vi "Dresden R2R Sputter 03.02.2018 IY24.vi"() -> ()   [LabVIEW 2009] (continued)
                                }
                                }
                                n17668 = local read "Semi"() -> (w26061:bool)
                                n17669 = Or(x=w26062, y=w26061) -> (x .or. y?=w26060:bool)
                                }
                                }
                                frame #1 {
                                }
                                }
                                }
                                frame #1 {
                                n17670 = local read "Semi"() -> (w26073:bool)
                                n17671 = case shown="False" w26073 {
                                frame #0 {
                                n17672 = local write "Ch2_PA7"(TRUE ("PA3")) -> ()
                                n17673 = Wait Until Next ms Multiple(millisecond multiple=u32 1000) -> ()  [unwired: 1 out]
                                }
                                frame #1 {
                                }
                                }
                                }
                                }
                              }
                              frame #1 {
                              }
                            }
                          }
                          frame #2 {
                            # "CLOSE BG-BV"
                            n17674 = local read "Semi"() -> (w26076:bool)
                            n17675 = case shown="False" w26076 {
                              frame #0 {
                                n17676 = stacked-sequence {
                                frame #0 {
                                n17677 = local read "Semi"() -> (w26077:bool)
                                n17678 = case shown="False" w26077 {
                                frame #0 {
                                n17679 = while {
                                i -> [w26084]
                                stop <- w26078 stop-if-true
                                n17680 = Greater?(x=w26084, y=50) -> (0:w26082:bool)
                                n17681 = case shown="True" w26082 {
                                frame #0 {
                                }
                                frame #1 {
                                n17682 = local write "Semi"(TRUE ("Semi")) -> ()
                                n17683 = local write "Error Message"("Start up process  cancelled\nbecause  BG-BV not closed.\nPlease check  BG-BV2 connections." ("Error Message")) -> ()
                                }
                                }
                                n17684 = local read "Ch2_Bg_bv_di"() -> (w26081:bool)
                                n17685 = case shown="True" w26081 {
                                tunnel: [TRUE FALSE] -> w26080
                                frame #0 {
                                }
                                frame #1 {
                                n17686 = Wait Until Next ms Multiple(millisecond multiple=u32 200) -> ()  [unwired: 1 out]
                                n17687 = local write "Ch2_Bg_bv_do"(FALSE ("Ch1_Tp_bv_do")) -> ()
                                }
                                }
                                n17688 = local read "Semi"() -> (w26079:bool)
                                n17689 = Or(x=w26080, y=w26079) -> (x .or. y?=w26078:bool)
                                }
                                }
                                frame #1 {
                                }
                                }
                                }
                                frame #1 {
                                n17690 = local read "Semi"() -> (w26091:bool)
                                n17691 = case shown="False" w26091 {
                                frame #0 {
                                n17692 = local write "Ch2_PA8"(TRUE ("PA3")) -> ()
                                n17693 = Wait Until Next ms Multiple(millisecond multiple=u32 1000) -> ()  [unwired: 1 out]
                                }
                                frame #1 {
                                }
                                }
                                }
                                }
                              }
                              frame #1 {
                              }
                            }
                          }
                          frame #3 {
                            # "CLOSE TP-BV"
                            n17694 = local read "Semi"() -> (w26094:bool)
                            n17695 = case shown="False" w26094 {
                              frame #0 {
                                n17696 = stacked-sequence {
                                frame #0 {
                                n17697 = local read "Semi"() -> (w26095:bool)
                                n17698 = case shown="False" w26095 {
                                frame #0 {
                                n17699 = while {
                                i -> [w26102]
                                stop <- w26096 stop-if-true
                                n17700 = Greater?(x=w26102, y=50) -> (0:w26100:bool)
                                n17701 = case shown="True" w26100 {
                                frame #0 {
                                }
                                frame #1 {
                                n17702 = local write "Semi"(TRUE ("Semi")) -> ()
                                n17703 = local write "Error Message"("Start up process  cancelled\nbecause  TP-BV not closed.\nPlease check  TP2-BV connections." ("Error Message")) -> ()
                                }
                                }
                                n17704 = local read "Ch2_Tp_bv_di"() -> (w26099:bool)
                                n17705 = case shown="True" w26099 {
                                tunnel: [TRUE FALSE] -> w26098
                                frame #0 {
                                }
                                frame #1 {
                                n17706 = Wait Until Next ms Multiple(millisecond multiple=u32 200) -> ()  [unwired: 1 out]
                                n17707 = local write "Ch2_Tp_bv_do"(FALSE ("Ch1_Tp_bv_do")) -> ()
                                }
                                }
                                n17708 = local read "Semi"() -> (w26097:bool)
                                n17709 = Or(x=w26098, y=w26097) -> (x .or. y?=w26096:bool)
                                }
                                }
                                frame #1 {
                                }
                                }
                                }
                                frame #1 {
                                n17710 = local read "Semi"() -> (w26109:bool)
                                n17711 = case shown="False" w26109 {
                                frame #0 {
                                n17712 = local write "Ch2_PA9"(TRUE ("PA5")) -> ()
                                n17713 = Wait Until Next ms Multiple(millisecond multiple=u32 1000) -> ()  [unwired: 1 out]
                                }
                                frame #1 {
                                }
                                }
                                }
                                }
                              }
                              frame #1 {
                              }
                            }
                          }
                          frame #4 {
                            # "False PL1-ATM"
                            n17714 = local read "Semi"() -> (w26112:bool)
                            n17715 = case shown="False" w26112 {
                              frame #0 {
                                n17716 = stacked-sequence {
                                frame #0 {
                                n17717 = local read "Semi"() -> (w26113:bool)
                                n17718 = case shown="False" w26113 {
                                frame #0 {
                                n17719 = local write "Ch2_Pl_atm_do"(FALSE ("Ch1_Pl_atm_do")) -> ()
                                }
                                frame #1 {
                                }
                                }
                                }
                                frame #1 {
                                n17720 = local read "Semi"() -> (w26115:bool)
                                n17721 = case shown="False" w26115 {
                                frame #0 {
                                n17722 = local write "Ch2_PA10"(TRUE ("PA3")) -> ()
                                n17723 = Wait Until Next ms Multiple(millisecond multiple=u32 1000) -> ()  [unwired: 1 out]
                                }
                                frame #1 {
                                }
                                }
                                }
                                }
                              }
                              frame #1 {
                              }
                            }
                          }
                          frame #5 {
                            # "STOP MP"
                            n17724 = local read "Semi"() -> (w26118:bool)
                            n17725 = case shown="False" w26118 {
                              frame #0 {
                                n17726 = stacked-sequence {
                                frame #0 {
                                n17727 = local read "Semi"() -> (w26119:bool)
                                n17728 = case shown="False" w26119 {
                                frame #0 {
                                n17729 = while {
                                i -> [w26126]
                                stop <- w26120 stop-if-true
                                n17730 = Greater?(x=w26126, y=50) -> (0:w26124:bool)
                                n17731 = case shown="True" w26124 {
                                frame #0 {
                                }
                                frame #1 {
                                n17732 = local write "Semi"(TRUE ("Semi")) -> ()
                                n17733 = local write "Error Message"("Start up process  cancelled\nbecause MP2 not stopped.\nPlease check MP2 connections." ("Error Message")) -> ()
                                }
                                }
                                n17734 = local read "Ch2_Mp_di"() -> (w26123:bool)
                                n17735 = case shown="True" w26123 {
                                tunnel: [TRUE FALSE] -> w26122
                                frame #0 {
                                }
                                frame #1 {
                                n17736 = Wait Until Next ms Multiple(millisecond multiple=u32 200) -> ()  [unwired: 1 out]
                                n17737 = local write "Ch2_Mp_do"(FALSE ("Ch1_Tp_bv_do")) -> ()
                                }
                                }
                                n17738 = local read "Semi"() -> (w26121:bool)
                                n17739 = Or(x=w26122, y=w26121) -> (x .or. y?=w26120:bool)
                                }
                                }
                                frame #1 {
                                }
                                }
                                }
                                frame #1 {
                                n17740 = local read "Semi"() -> (w26133:bool)
                                n17741 = case shown="False" w26133 {
                                frame #0 {
                                n17742 = local write "Ch2_PA11"(TRUE ("PA3")) -> ()
                                n17743 = Wait Until Next ms Multiple(millisecond multiple=u32 1000) -> ()  [unwired: 1 out]
                                }
                                frame #1 {
                                }
                                }
                                }
                                }
                              }
                              frame #1 {
                              }
                            }
                          }
                          frame #6 {
                            # "OPEN PL-VBV"
                            n17744 = local read "Semi"() -> (w26136:bool)
                            n17745 = case shown="False" w26136 {
                              frame #0 {
                                n17746 = stacked-sequence {
                                frame #0 {
                                n17747 = local read "Semi"() -> (w26137:bool)
                                n17748 = case shown="False" w26137 {
                                frame #0 {
                                n17749 = while {
                                i -> [w26144]
                                stop <- w26139 stop-if-true
                                n17750 = Greater?(x=w26144, y=50) -> (0:w26142:bool)
                                n17751 = case shown="True" w26142 {
                                frame #0 {
                                }
                                frame #1 {
                                n17752 = local write "Semi"(TRUE ("Semi")) -> ()
                                n17753 = local write "Error Message"("Start up process  cancelled\nbecause  PL-VBV not opened.\nPlease check PL-VBV2 connections." ("Error Message")) -> ()
                                }
                                }
                                n17754 = local read "Ch2_Pl_atm_di"() -> (w26138:bool)
                                n17755 = case shown="False" w26138 {
                                tunnel: [w26146 TRUE] -> w26141
                                frame #0 {
                                n17756 = local read "Ch2_Pl_vbv_di"() -> (w26145:bool)
                                n17757 = case shown="False" w26145 {
                                tunnel: [FALSE TRUE] -> w26146
                                frame #0 {
                                n17758 = Wait Until Next ms Multiple(millisecond multiple=u32 200) -> ()  [unwired: 1 out]
                                n17759 = local write "Ch2_Pl_vbv_do"(TRUE ("Ch1_Tp_bv_do")) -> ()
                                }
                                frame #1 {
                                }
                                }
                                }
                                frame #1 {
                                }
                                }
                                n17760 = local read "Semi"() -> (w26140:bool)
                                n17761 = Or(x=w26141, y=w26140) -> (x .or. y?=w26139:bool)
                                }
                                }
                                frame #1 {
                                }
                                }
                                }
                                frame #1 {
                                n17762 = local read "Semi"() -> (w26154:bool)
                                n17763 = case shown="False" w26154 {
                                frame #0 {
                                n17764 = local write "Ch2_PA12"(TRUE ("PA3")) -> ()
                                n17765 = Wait Until Next ms Multiple(millisecond multiple=u32 1000) -> ()  [unwired: 1 out]
                                }
                                frame #1 {
                                }
                                }
                                }
                                }
                              }
                              frame #1 {
                              }
                            }
                          }
                          frame #7 {
                            # "CHECK PL-PRESSURE"
                            n17766 = local read "Semi"() -> (w26157:bool)
                            n17767 = case shown="False" w26157 {
                              frame #0 {
                                n17768 = stacked-sequence {
                                frame #0 {
                                n17769 = local read "Semi"() -> (w26158:bool)
                                n17770 = case shown="False" w26158 {
                                frame #0 {
                                n17771 = while {
                                i -> [w26165]
                                stop <- w26160 stop-if-true
                                n17772 = Greater?(x=w26165, y=50) -> (0:w26163:bool)
                                n17773 = case shown="True" w26163 {
                                frame #0 {
                                }
                                frame #1 {
                                n17774 = local write "Semi"(TRUE ("Semi")) -> ()
                                n17775 = local write "Error Message"("Start up process  cancelled\nbecause  PL-ATM not opened.\nPlease check PL-ATM2 connections." ("Error Message")) -> ()
                                }
                                }
                                n17776 = local read "Ch2_Pl_atm_di"() -> (w26159:bool)
                                n17777 = case shown="True" w26159 {
                                tunnel: [FALSE TRUE] -> w26162
                                frame #0 {
                                }
                                frame #1 {
                                n17778 = Wait Until Next ms Multiple(millisecond multiple=u32 500) -> ()  [unwired: 1 out]
                                }
                                }
                                n17779 = local read "Semi"() -> (w26161:bool)
                                n17780 = Or(x=w26162, y=w26161) -> (x .or. y?=w26160:bool)
                                }
                                }
                                frame #1 {
                                }
                                }
                                }
                                frame #1 {
                                n17781 = local read "Semi"() -> (w26171:bool)
                                n17782 = case shown="False" w26171 {
                                frame #0 {
                                n17783 = local write "Ch2_PA13"(TRUE ("PA3")) -> ()
                                n17784 = Wait Until Next ms Multiple(millisecond multiple=u32 1000) -> ()  [unwired: 1 out]
                                }
                                frame #1 {
                                }
                                }
                                }
                                }
                              }
                              frame #1 {
                              }
                            }
                          }
                          frame #8 {
                            # "False CH-ATM"
                            n17785 = local read "Semi"() -> (w26174:bool)
                            n17786 = case shown="False" w26174 {
                              frame #0 {
                                n17787 = stacked-sequence {
                                frame #0 {
                                n17788 = local read "Semi"() -> (w26175:bool)
                                n17789 = case shown="False" w26175 {
                                frame #0 {
                                n17790 = local write "Ch2_Ch_atm_do"(FALSE ("Ch1_Pl_atm_do")) -> ()
                                }
                                frame #1 {
                                }
                                }
                                }
                                frame #1 {
                                n17791 = local read "Semi"() -> (w26177:bool)
                                n17792 = case shown="False" w26177 {
                                frame #0 {
                                n17793 = local write "Ch2_PA14"(TRUE ("PA3")) -> ()
                                n17794 = Wait Until Next ms Multiple(millisecond multiple=u32 1000) -> ()  [unwired: 1 out]
                                }
                                frame #1 {
                                }
                                }
                                }
                                }
                              }
                              frame #1 {
                              }
                            }
                          }
                          frame #9 {
                            # "OPEN PC-BV"
                            n17795 = local read "Semi"() -> (w26180:bool)
                            n17796 = case shown="False" w26180 {
                              frame #0 {
                                n17797 = stacked-sequence {
                                frame #0 {
                                n17798 = local read "Semi"() -> (w26181:bool)
                                n17799 = case shown="False" w26181 {
                                frame #0 {
                                n17800 = stacked-sequence {
                                frame #0 {
                                n17801 = local read "Semi"() -> (w26182:bool)
                                n17802 = case shown="False" w26182 {
                                frame #0 {
                                n17803 = local write "Pc_bv2_auto_open"(TRUE ("Tp1_auto_start")) -> ()
                                }
                                frame #1 {
                                }
                                }
                                }
                                frame #1 {
                                n17804 = local read "Semi"() -> (w26184:bool)
                                n17805 = case shown="False" w26184 {
                                frame #0 {
                                n17806 = Wait (ms)(milliseconds to wait=u32 1000) -> ()  [unwired: 1 out]
                                }
                                frame #1 {
                                }
                                }
                                }
                                frame #2 {
                                n17807 = local read "Semi"() -> (w26186:bool)
                                n17808 = case shown="False" w26186 {
                                frame #0 {
                                n17809 = while {
                                i -> [w26192]
                                stop <- w26188 stop-if-true
                                n17810 = local read "Pc_bv_opened_ch2"() -> (w26190:bool)
                                n17811 = Greater?(x=w26192, y=120) -> (0:w26191:bool)
                                n17812 = local read "Semi"() -> (w26189:bool)
                                n17813 = Compound Arithmetic op=OR(w26189, w26190, w26191) -> (w26188:bool)
                                n17814 = Wait (ms)(milliseconds to wait=u32 500) -> ()  [unwired: 1 out]
                                }
                                }
                                frame #1 {
                                }
                                }
                                }
                                frame #3 {
                                n17815 = local read "Semi"() -> (w26194:bool)
                                n17816 = case shown="False" w26194 {
                                frame #0 {
                                n17817 = local read "Pc_bv_opened_ch2"() -> (w26195:bool)
                                n17818 = case shown="False" w26195 {
                                frame #0 {
                                n17819 = local write "Pc_bv2_auto_open"(TRUE ("Pc_bv1_auto_open")) -> ()
                                }
                                frame #1 {
                                }
                                }
                                }
                                frame #1 {
                                }
                                }
                                }
                                frame #4 {
                                n17820 = local read "Semi"() -> (w26197:bool)
                                n17821 = case shown="False" w26197 {
                                frame #0 {
                                n17822 = local read "Pc_bv_opened_ch2"() -> (w26198:bool)
                                n17823 = case shown="False" w26198 {
                                frame #0 {
                                n17824 = Wait (ms)(milliseconds to wait=u32 1000) -> ()  [unwired: 1 out]
                                }
                                frame #1 {
                                }
                                }
                                }
                                frame #1 {
                                }
                                }
                                }
                                frame #5 {
                                n17825 = local read "Semi"() -> (w26200:bool)
                                n17826 = case shown="False" w26200 {
                                frame #0 {
                                n17827 = while {
                                i -> [w26206]
                                stop <- w26202 stop-if-true
                                n17828 = local read "Pc_bv_opened_ch2"() -> (w26204:bool)
                                n17829 = Greater?(x=w26206, y=120) -> (0:w26205:bool)
                                n17830 = local read "Semi"() -> (w26203:bool)
                                n17831 = Compound Arithmetic op=OR(w26203, w26204, w26205) -> (w26202:bool)
                                n17832 = Wait (ms)(milliseconds to wait=u32 500) -> ()  [unwired: 1 out]
                                }
                                }
                                frame #1 {
                                }
                                }
                                }
                                frame #6 {
                                n17833 = local read "Semi"() -> (w26208:bool)
                                n17834 = case shown="False" w26208 {
                                frame #0 {
                                n17835 = local read "Pc_bv_opened_ch2"() -> (w26209:bool)
                                n17836 = case shown="False" w26209 {
                                frame #0 {
                                n17837 = local write "Error Message"("Start up process  cancelled\nbecause  PC-BV not opened.\nPlease check PC-BV2 connections." ("Error Message")) -> ()
                                n17838 = Wait (ms)(milliseconds to wait=u32 1000) -> ()  [unwired: 1 out]
                                }
                                frame #1 {
                                }
                                }
                                }
                                frame #1 {
                                }
                                }
                                }
                                }
                                }
                                frame #1 {
                                }
                                }
                                }
                                frame #1 {
                                n17839 = local read "Semi"() -> (w26212:bool)
                                n17840 = case shown="False" w26212 {
                                frame #0 {
                                n17841 = local write "Ch2_PA15"(TRUE ("PA3")) -> ()
                                n17842 = Wait Until Next ms Multiple(millisecond multiple=u32 1000) -> ()  [unwired: 1 out]
                                }
                                frame #1 {
                                }
                                }
                                }
                                }
                              }
                              frame #1 {
                              }
                            }
                          }
                          frame #10 {
                            # "OPEN CH-VBV"
                            n17843 = local read "Semi"() -> (w26215:bool)
                            n17844 = case shown="False" w26215 {
                              frame #0 {
                                n17845 = stacked-sequence {
                                frame #0 {
                                n17846 = local read "Semi"() -> (w26216:bool)
                                n17847 = case shown="False" w26216 {
                                frame #0 {
                                n17848 = while {
                                i -> [w26223]
                                stop <- w26218 stop-if-true
                                n17849 = Greater?(x=w26223, y=50) -> (0:w26221:bool)
                                n17850 = case shown="True" w26221 {
                                frame #0 {
                                }
                                frame #1 {
                                n17851 = local write "Semi"(TRUE ("Semi")) -> ()
                                n17852 = local write "Error Message"("Start up process  cancelled\nbecause  CH-VBV not opened.\nPlease check  CH2-VBV connections." ("Error Message")) -> ()
                                }
                                }
                                n17853 = local read "Ch2_Ch_atm_di"() -> (w26217:bool)
                                n17854 = case shown="False" w26217 {
                                tunnel: [w26224 TRUE] -> w26220
                                frame #0 {
                                n17855 = local read "Ch2_Ch_vbv_di"() -> (w26225:bool)
                                n17856 = case shown="False" w26225 {
                                tunnel: [FALSE TRUE] -> w26224
                                frame #0 {
                                n17857 = local write "Ch2_Ch_vbv_do"(TRUE ("Ch1_Tp_bv_do")) -> ()
                                n17858 = Wait Until Next ms Multiple(millisecond multiple=u32 200) -> ()  [unwired: 1 out]
                                }
                                frame #1 {
                                }
                                }
                                }
                                frame #1 {
                                }
                                }
                                n17859 = local read "Semi"() -> (w26219:bool)
                                n17860 = Or(x=w26220, y=w26219) -> (x .or. y?=w26218:bool)
                                }
                                }
                                frame #1 {
                                }
                                }
                                }
                                frame #1 {
                                n17861 = local read "Semi"() -> (w26233:bool)
                                n17862 = case shown="False" w26233 {
                                frame #0 {
                                n17863 = local write "Ch2_PA16"(TRUE ("PA3")) -> ()
                                n17864 = Wait Until Next ms Multiple(millisecond multiple=u32 1000) -> ()  [unwired: 1 out]
                                }
                                frame #1 {
                                }
                                }
                                }
                                }
                              }
                              frame #1 {
                              }
                            }
                          }
                          frame #11 {
                            # "OPEN/CLOSE TRNS GV-BP2"
                            n17865 = local read "Semi"() -> (w26236:bool)
                            n17866 = case shown="False" w26236 {
                              frame #0 {
                                n17867 = stacked-sequence {
                                frame #0 {
                                n17868 = local read "Semi"() -> (w26237:bool)
                                n17869 = case shown="False" w26237 {
                                frame #0 {
                                n17870 = while {
                                i -> [w26246]
                                stop <- w26241 stop-if-true
                                n17871 = Greater?(x=w26246, y=800) -> (0:w26244:bool)
                                n17872 = case shown="True" w26244 {
                                frame #0 {
                                }
                                frame #1 {
                                n17873 = local read "Ch3_pressure"() -> (w26266:dbl)
                                n17874 = Less?(x=w26266, y=1) -> (x < y?=w26265:bool)
                                n17875 = case shown="True" w26265 {
                                frame #0 {
                                n17876 = local write "Error Message"("Start up process  cancelled\nbecause \n Trns GV-BP2 not closed.\nPlease check \nTrns GV-BP2 connections." ("Error Message")) -> ()
                                }
                                frame #1 {
                                n17877 = local write "Error Message"("Start up process  cancelled\nbecause \n Trns GV-BP2 not opened.\nPlease check \nTrns GV-BP2 connections." ("Error Message")) -> ()
                                }
                                }
                                n17878 = local write "Semi"(TRUE ("Semi")) -> ()
                                }
                                }
                                n17879 = local read "Ch3_pressure"() -> (w26240:dbl)
                                n17880 = Less?(x=w26240, y=1) -> (x < y?=w26238:bool)
                                n17881 = case shown="True" w26238 {
                                tunnel: [w26248 w26256] -> w26243
                                frame #0 {
                                n17882 = local read "Ch1_Trns_gv_bp2_di"() -> (w26247:bool)
                                n17883 = case shown="True" w26247 {
                                tunnel: [TRUE FALSE] -> w26248
                                frame #0 {
                                }
                                frame #1 {
                                n17884 = local write "Ch1_Trns_gv_bp2_do"(FALSE ("Ch1_Tp_bv_do")) -> ()
                                n17885 = Wait Until Next ms Multiple(millisecond multiple=u32 200) -> ()  [unwired: 1 out]
                                }
                                }
                                }
                                frame #1 {
                                n17886 = local read "Ch2_pressure"() -> (w26255:dbl)
                                n17887 = Greater Or Equal?(x=w26255, y=700.0) -> (x >= y?=w26253:bool)
                                n17888 = case shown="True" w26253 {
                                tunnel: [FALSE w26260] -> w26256
                                frame #0 {
                                n17889 = Wait Until Next ms Multiple(millisecond multiple=u32 500) -> ()  [unwired: 1 out]
                                }
                                frame #1 {
                                n17890 = local read "Ch2_trns_gv_bp2_di"() -> (w26259:bool)
                                n17891 = case shown="False" w26259 {
                                tunnel: [FALSE TRUE] -> w26260
                                frame #0 {
                                n17892 = local write "Ch2_trns_gv_bp2_do"(TRUE ("Ch1_Tp_bv_do")) -> ()
                                n17893 = Wait Until Next ms Multiple(millisecond multiple=u32 200) -> ()  [unwired: 1 out]
                                }
                                frame #1 {
                                }
                                }
                                }
                                }
                                }
                                }
                                n17894 = local read "Semi"() -> (w26242:bool)
                                n17895 = Or(x=w26243, y=w26242) -> (x .or. y?=w26241:bool)
                                }
                                }
                                frame #1 {
                                }
                                }
                                }
                                frame #1 {
                                n17896 = local read "Semi"() -> (w26271:bool)
                                n17897 = case shown="False" w26271 {
                                frame #0 {
                                n17898 = local write "Ch2_PA17"(TRUE ("PA3")) -> ()
                                n17899 = Wait Until Next ms Multiple(millisecond multiple=u32 1000) -> ()  [unwired: 1 out]
                                }
                                frame #1 {
                                }
                                }
                                }
                                }
                              }
                              frame #1 {
                              }
                            }
                          }
                          frame #12 {
                            # "OPEN/CLOSE TRNS GV-BP"
                            n17900 = local read "Semi"() -> (w26274:bool)
                            n17901 = case shown="False" w26274 {
                              frame #0 {
                                n17902 = stacked-sequence {
                                frame #0 {
                                n17903 = local read "Semi"() -> (w26275:bool)
                                n17904 = case shown="False" w26275 {
                                frame #0 {
                                n17905 = while {
                                i -> [w26284]
                                stop <- w26279 stop-if-true
                                n17906 = Greater?(x=w26284, y=800) -> (0:w26282:bool)
                                n17907 = case shown="True" w26282 {
                                frame #0 {
                                }
                                frame #1 {
                                n17908 = local read "Ch1_pressure"() -> (w26304:dbl)
                                n17909 = Less?(x=w26304, y=1) -> (x < y?=w26303:bool)
                                n17910 = case shown="False" w26303 {
                                frame #0 {
                                n17911 = local write "Error Message"("Start up process  cancelled\nbecause  \nTrns GV-BP not closed.\nPlease check \nTrns GV-BP connections." ("Error Message")) -> ()
                                }
                                frame #1 {
                                n17912 = local write "Error Message"("Start up process  cancelled\nbecause \n Trns GV-BP not opened.\nPlease check \nTrns GV-BP connections." ("Error Message")) -> ()
                                }
                                }
                                n17913 = local write "Semi"(TRUE ("Semi")) -> ()
                                }
                                }
                                n17914 = local read "Ch1_pressure"() -> (w26278:dbl)
                                n17915 = Less?(x=w26278, y=1) -> (x < y?=w26276:bool)
                                n17916 = case shown="True" w26276 {
                                tunnel: [w26286 w26294] -> w26281
                                frame #0 {
                                n17917 = local read "Ch2_trns_gv_bp_di"() -> (w26285:bool)
                                n17918 = case shown="True" w26285 {
                                tunnel: [TRUE FALSE] -> w26286
                                frame #0 {
                                }
                                frame #1 {
                                n17919 = local write "Ch2_trns_gv_bp_do"(FALSE ("Ch1_Tp_bv_do")) -> ()
                                n17920 = Wait Until Next ms Multiple(millisecond multiple=u32 200) -> ()  [unwired: 1 out]
                                }
                                }
                                }
                                frame #1 {
                                n17921 = local read "Ch2_pressure"() -> (w26292:dbl)
                                n17922 = Greater Or Equal?(x=w26292, y=700.0) -> (x >= y?=w26291:bool)
                                n17923 = case shown="True" w26291 {
                                tunnel: [FALSE w26298] -> w26294
                                frame #0 {
                                n17924 = Wait Until Next ms Multiple(millisecond multiple=u32 500) -> ()  [unwired: 1 out]
                                }
                                frame #1 {
                                n17925 = local read "Ch2_trns_gv_bp_di"() -> (w26297:bool)
                                n17926 = case shown="False" w26297 {
                                tunnel: [FALSE TRUE] -> w26298
                                frame #0 {
                                n17927 = local write "Ch2_trns_gv_bp_do"(TRUE ("Ch1_Tp_bv_do")) -> ()
                                n17928 = Wait Until Next ms Multiple(millisecond multiple=u32 200) -> ()  [unwired: 1 out]
                                }
                                frame #1 {
                                }
                                }
                                }
                                }
                                }
                                }
                                n17929 = local read "Semi"() -> (w26280:bool)
                                n17930 = Or(x=w26281, y=w26280) -> (x .or. y?=w26279:bool)
                                }
                                }
                                frame #1 {
                                }
                                }
                                }
                                frame #1 {
                                n17931 = local read "Semi"() -> (w26309:bool)
                                n17932 = case shown="False" w26309 {
                                frame #0 {
                                n17933 = local write "Ch2_PA18"(TRUE ("PA3")) -> ()
                                n17934 = Wait Until Next ms Multiple(millisecond multiple=u32 1000) -> ()  [unwired: 1 out]
                                }
                                frame #1 {
                                }
                                }
                                }
                                }
                              }
                              frame #1 {
                              }
                            }
                          }
                          frame #13 {
                            # "CHECK CH-ATM"
                            n17935 = local read "Semi"() -> (w26312:bool)
                            n17936 = case shown="False" w26312 {
                              frame #0 {
                                n17937 = stacked-sequence {
                                frame #0 {
                                n17938 = local read "Semi"() -> (w26313:bool)
                                n17939 = case shown="False" w26313 {
                                frame #0 {
                                n17940 = while {
                                i -> [w26320]
                                stop <- w26315 stop-if-true
                                n17941 = Greater?(x=w26320, y=1200) -> (0:w26318:bool)
                                n17942 = case shown="True" w26318 {
                                frame #0 {
                                }
                                frame #1 {
                                n17943 = local write "Semi"(TRUE ("Semi")) -> ()
                                n17944 = local write "Error Message"("Start up process  cancelled\nbecause  CH-ATM not opened.\nPlease check CH-ATM connections." ("Error Message")) -> ()
                                }
                                }
                                n17945 = local read "Ch2_Ch_atm_di"() -> (w26314:bool)
                                n17946 = case shown="False" w26314 {
                                tunnel: [FALSE TRUE] -> w26317
                                frame #0 {
                                n17947 = Wait Until Next ms Multiple(millisecond multiple=u32 500) -> ()  [unwired: 1 out]
                                }
                                frame #1 {
                                }
                                }
                                n17948 = local read "Semi"() -> (w26316:bool)
                                n17949 = Or(x=w26317, y=w26316) -> (x .or. y?=w26315:bool)
                                }
                                }
                                frame #1 {
                                }
                                }
                                }